vi "datatakersync.vi"() -> ()   [LabVIEW 2013]
doc: "This example demonstrates how to acquire a single buffer of voltage measurements using a DAQmx device.\n\nFor instructions on how to connect your signals to the DAQ device, refer to your device documentation."
uses:
  <vilib>/userdefined/High Color/nirio_resource_hc.ctl
  <vilib>/Utility/error.llb/DialogType.ctl
  <vilib>/FPGAPlugInAG/PCIe-7841R/niLvFpga_Open_PCIe-7841R.vi
  <vilib>/DAQmx/create/channels.llb/DAQmx Create Channel (AI-Voltage-Basic).vi
  <vilib>/DAQmx/configure/timing.llb/DAQmx Timing (Sample Clock).vi
  <vilib>/DAQmx/configure/trigger.llb/DAQmx Start Trigger (Digital Edge).vi
  <vilib>/rvi/interface/nirviOpenFPGA/nirviOpenFPGA.xnode
  fpga/MultiChannelFeed_FPGATarget2_feedbackcooling(_T5hmXv3JUos.lvbitx
  <resource>/objmgr/daqmx.rc
panel:
  in  "sweep time (S)":ext=10.0 format="%.2f"
  in  "sweep stop (Hz)":ext=200.0
  in  "sweep start (Hz)":ext=1.0
  in  "chirp?":bool
  in  "stop (F)":ext=200.0
  in  "start (F)":ext=10.0
  in  "Number of F Steps":i32=20
  in  "dc offset?":bool=TRUE
  in  "volt_div":dbl=200.0
  in  "Set synth?":bool=TRUE
  in  "stop (V)":ext=2.5
  in  "start (V)":ext=2.5
  in  "Number of V Steps":i32=1
  out "error out":errorcluster
  in  "Physical Channel (drive signals)":tag="Dev5/ai0"
  out "Curr threshold":dbl
  in  "Stop threshold":dbl=0.05
  in  "Stop flashing below thresh":bool
  out "Pirani pressure (mbar)":string="0000\r\n"
  out "CC read error":errorcluster={"status"=FALSE, "code"=1073676294, "source"="VISA Read in read_pressure(SubVI).vi->hdf5(SubVI).vi->datataker.vi"}
  out "CC pressure (mbar)":string="4."
  out "Pirani read error":errorcluster={"status"=FALSE, "code"=1073676294, "source"="VISA Read in read_pressure(SubVI).vi->hdf5(SubVI).vi->datataker.vi"}
  in  "# Pulses":i32=3
  in  "Output channel (for flashing)":tag="Dev4/ao0"
  in  "Number of cyles\nbetween flashes":i32=3
  in  "Flash lamp?":bool
  in  "File base name":string="5e-7mbar_xyzcool"
  in  "Delay time between files(s)":dbl caption="Delay Time (s)"
  in  "Num files":i32=100000
  out "Temps (C):":dbl[](array[numeric])=[24.1, 24.6]
  in  "VISA Refnum in":refnum<visa-resource-name>="GPIB0::19::INSTR"
  in  "RIO Device":T1="RIO0::INSTR"
  in  "Directory path":path=path "D:/Data/20140623/Bead1/freq_sweep_finer"
  out "Waveform Graph":dbl[][](graph)
  in  "Number of Samples":i32=500000
  in  "Sample Rate":dbl=5000.0
  in  "Sample Clock Source":tag="/Dev2/PXI_Clk10"
  in  "Terminal Configuration":i32(ring)=-1 items=["default"=-1, "RSE"=10083, "NRSE"=10078, "Differential"=10106, "Pseudodifferential"=12529]
  in  "Max Voltage":dbl=10.0
  in  "Physical Channels (Position signals)":tag="Dev2/ai0:7"
  out "Actual Sample Rate":dbl=5000.0 format="%0.2f"
  # "Channel Settings"
  # "Acquired Data"
  # "Timing Settings"
  # "Flash Lamp Settings"
  # "Pressures and Temperatures"
  # "Logging Settings"
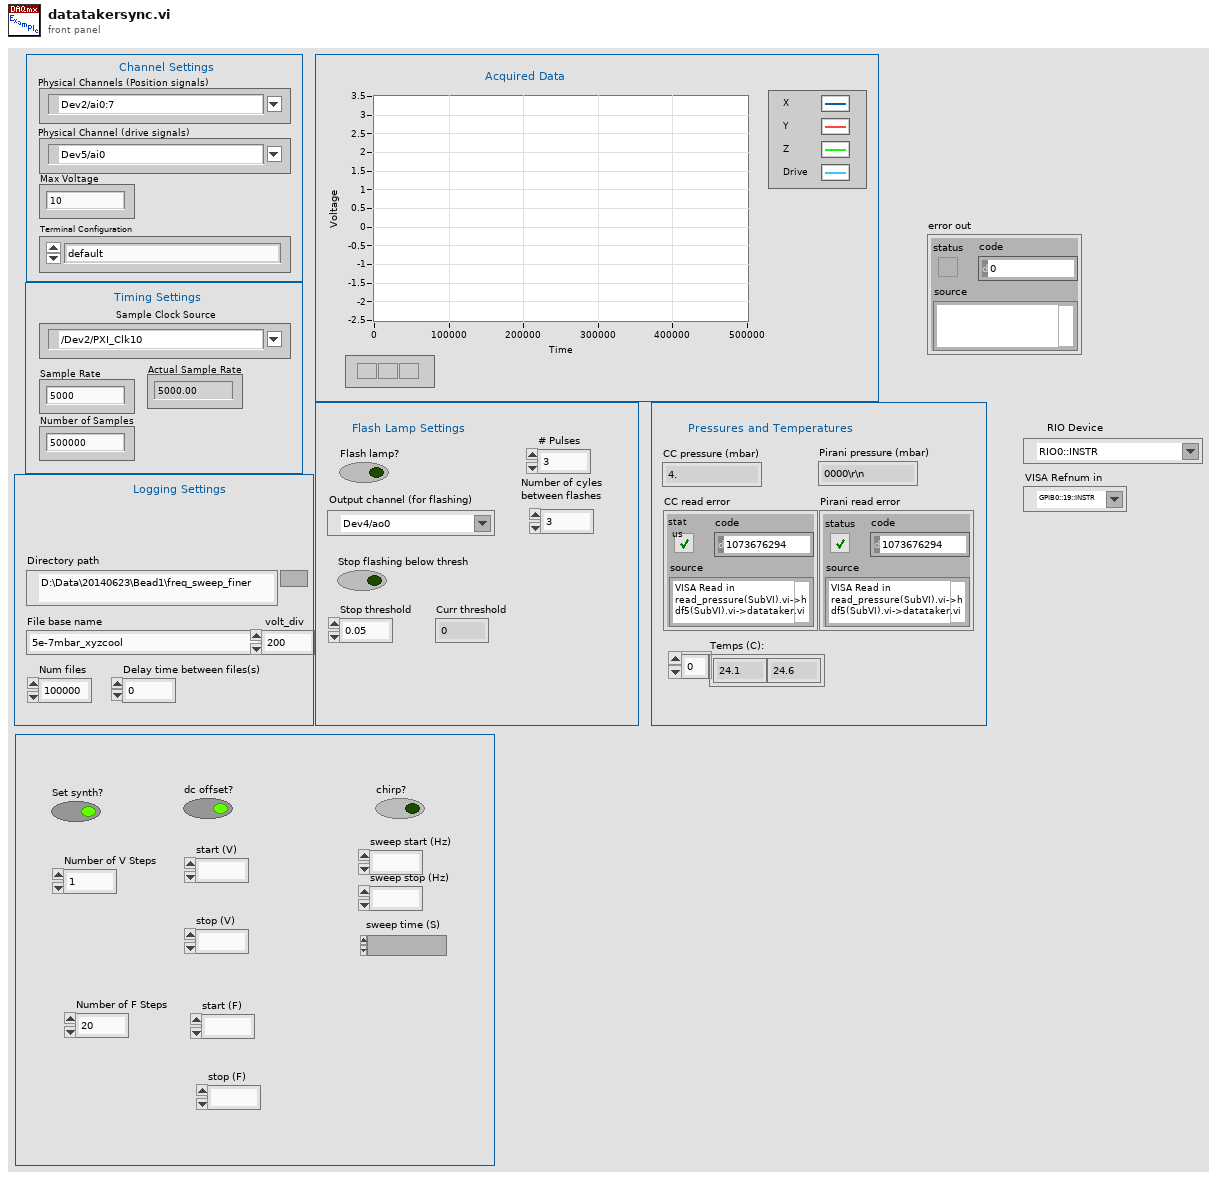
[diagram p1: front panel]
types:
  T1 = typedef "nirio_resource_hc.ctl" = tag
  T2 = typedef "DialogType.ctl" = u16
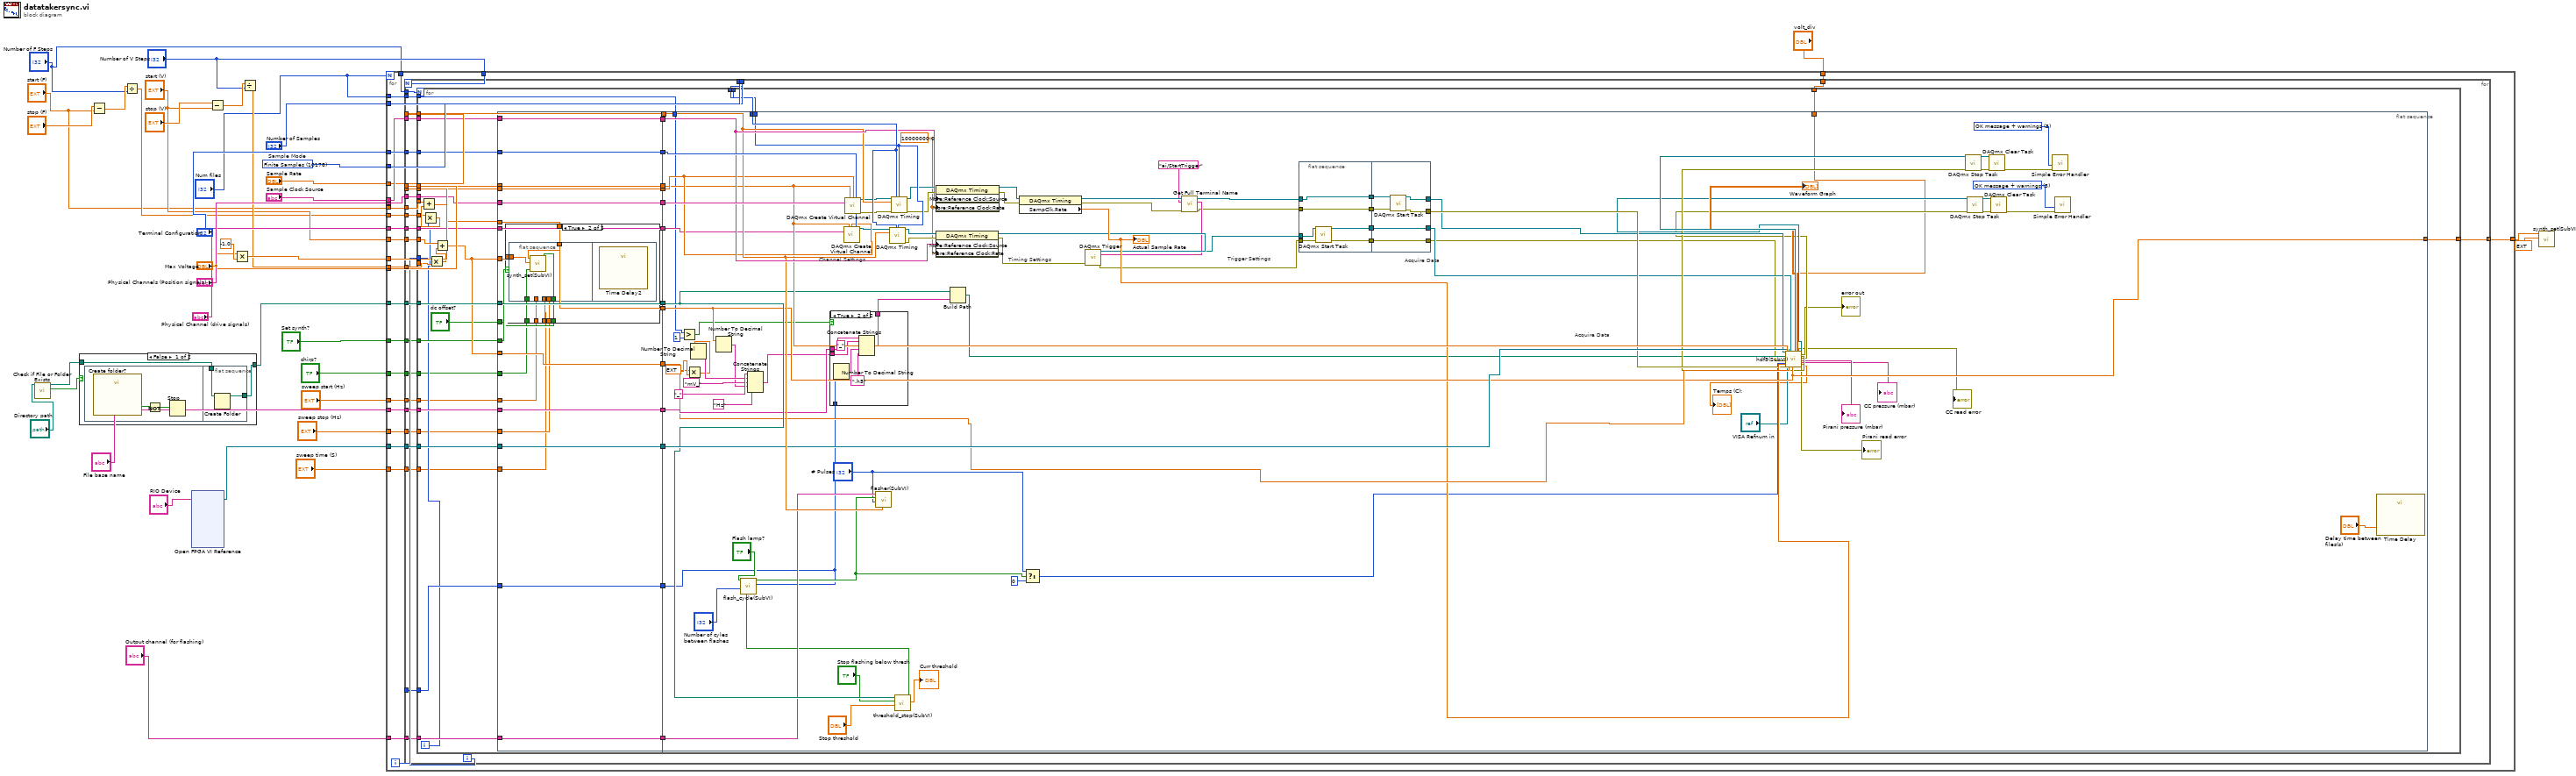
[diagram p0: block diagram]
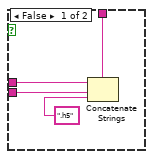
[diagram p3: hidden frame]
diagram:
  w37 = 10178 items=["Finite Samples"=10178, "Continuous Samples"=10123, "Hardware Timed Single Point"=12522]  # Sample Mode
  n1 = call <vilib>:"Check if File or Folder Exists.vi"("path"="Directory path") -> ("file or folder exists?"=w25:bool, "dup path"=w24:path)  [unwired: 8 in, 1 out]
  n2 = case shown="False" w25 {
    tunnel: w24 -> [w39 w44]
    tunnel: [w38 w44] -> w23
    frame False {
      n3 = flat-sequence {
        tunnel: w39 -> [w43]
        tunnel: [w42] -> w38
        frame #0 {
          n4 = call "Create folder?"() -> ("OK"=w41:bool)  [unwired: 18 in, 1 out]
          n5 = Not(x=w41) -> (.not. x?=w40:bool)
          n6 = Stop(stop? (T)=w40) -> ()
        }
        frame #1 {
          n7 = Create Folder(path (use dialog)=w43) -> (created path=w42:path)  [unwired: 2 in, 2 out]
        }
      }
    }
    frame True {
    }
  }
  n8 = Subtract(x="stop (F)", y="start (F)") -> (x-y=w9:ext)
  n9 = Divide(x=w9, y="Number of F Steps") -> (x/y=w8:ext)
  n10 = xnode "Open FPGA VI Reference"("resource name"="RIO Device") -> ("FPGA VI Reference Out"=w27:refnum<k20>)  [unwired: 1 in, 1 out]
  n11 = Subtract(x="stop (V)", y="start (V)") -> (x-y=w18:ext)
  n12 = Multiply(x="Max Voltage", y=-1.0) -> (x*y=w30:dbl)
  n13 = Divide(x=w18, y="Number of V Steps") -> (x/y=w16:ext)
  n14 = for {
    N: "Num files" -> [_]
    tunnel: w37 -> [w72]
    tunnel: "Physical Channels (Position signals)" -> [w71]
    tunnel: "Terminal Configuration" -> [w70]
    tunnel: "Sample Clock Source" -> [w69]
    tunnel: "Sample Rate" -> [w68]
    tunnel: "Number of Samples" -> [w67]
    tunnel: w30 -> [w66]
    tunnel: "Max Voltage" -> [w65]
    tunnel: w27 -> [w64]
    tunnel: w23 -> [w63]
    tunnel: "File base name" -> [w62]
    tunnel: "Output channel (for flashing)" -> [w61]
    tunnel: "Physical Channel (drive signals)" -> [w60]
    tunnel: "Number of V Steps" -> [w59]
    tunnel: w16 -> [w58]
    tunnel: "start (V)" -> [w57]
    tunnel: [w56] -> w6
    tunnel: "Num files" -> [w54]
    tunnel: "Set synth?" -> [w53]
    tunnel: "volt_div" -> [w52]
    tunnel: w8 -> [w51]
    tunnel: "start (F)" -> [w50]
    tunnel: "Number of F Steps" -> [w49]
    tunnel: "chirp?" -> [w48]
    tunnel: "sweep start (Hz)" -> [w47]
    tunnel: "sweep stop (Hz)" -> [w46]
    tunnel: "sweep time (S)" -> [w45]
    i -> [w55]
    n15 = for {
      N: w59 -> [_]
      tunnel: w72 -> [w100]
      tunnel: w71 -> [w99]
      tunnel: w70 -> [w98]
      tunnel: w69 -> [w97]
      tunnel: w68 -> [w96]
      tunnel: w67 -> [w95]
      tunnel: w66 -> [w94]
      tunnel: w65 -> [w93]
      tunnel: w64 -> [w92]
      tunnel: w63 -> [w91]
      tunnel: w62 -> [w90]
      tunnel: w61 -> [w89]
      tunnel: w60 -> [w88]
      tunnel: w58 -> [w87]
      tunnel: w57 -> [w86]
      tunnel: [w85] -> w56
      tunnel: w55 -> [w83]
      tunnel: w54 -> [w82]
      tunnel: w53 -> [w81]
      tunnel: w52 -> [w80]
      tunnel: w51 -> [w79]
      tunnel: w50 -> [w78]
      tunnel: w49 -> [w77]
      tunnel: w48 -> [w76]
      tunnel: w47 -> [w75]
      tunnel: w46 -> [w74]
      tunnel: w45 -> [w73]
      i -> [w84]
      n16 = for {
        N: w77 -> [_]
        tunnel: w100 -> [w133]
        tunnel: w99 -> [w132]
        tunnel: w98 -> [w131]
        tunnel: w97 -> [w130]
        tunnel: w96 -> [w129]
        tunnel: w95 -> [w128]
        tunnel: w94 -> [w127]
        tunnel: w93 -> [w126]
        tunnel: w92 -> [w125]
        tunnel: w91 -> [w124]
        tunnel: w90 -> [w123]
        tunnel: w89 -> [w122]
        tunnel: w88 -> [w121]
        tunnel: w87 -> [w120]
        tunnel: w86 -> [w118]
        tunnel: [w116] -> w85
        tunnel: w84 -> [w115]
        tunnel: w83 -> [w114]
        tunnel: w82 -> [w113]
        tunnel: w81 -> [w112]
        tunnel: w80 -> [w111]
        tunnel: w79 -> [w107]
        tunnel: w78 -> [w106]
        tunnel: w76 -> [w104]
        tunnel: w75 -> [w103]
        tunnel: w74 -> [w102]
        tunnel: w73 -> [w101]
        i -> [w105]
        n17 = Multiply(x=w107, y=w105) -> (x*y=w108:ext)
        n18 = Add(x=w106, y=w108) -> (x+y=w109:ext)
        n19 = Multiply(x=w115, y=w120) -> (x*y=w119:ext)
        n20 = Add(x=w118, y=w119) -> (x+y=w117:ext)
        n21 = flat-sequence {
          tunnel: w121 -> [w157]
          tunnel: w122 -> [w158]
          tunnel: w123 -> [w159]
          tunnel: w124 -> [w160]
          tunnel: w125 -> [w161]
          tunnel: w126 -> [w162]
          tunnel: w127 -> [w163]
          tunnel: w130 -> [w164]
          tunnel: w131 -> [w165]
          tunnel: w132 -> [w166]
          tunnel: [w166] -> w146
          tunnel: [w165] -> w145
          tunnel: [w164] -> w144
          tunnel: [w163] -> w143
          tunnel: [w162] -> w142
          tunnel: [w161] -> w141
          tunnel: [w160] -> w140
          tunnel: [w159] -> w139
          tunnel: [w158] -> w138
          tunnel: [w157] -> w137
          tunnel: w109 -> [w155]
          tunnel: w117 -> [w156]
          tunnel: [w155] -> w136
          tunnel: w117 -> [w154]
          tunnel: [w154] -> w135
          tunnel: w114 -> [w153]
          tunnel: [w153] -> w134
          tunnel: w112 -> [w152]
          tunnel: "dc offset?" -> [w151]
          tunnel: w104 -> [w150]
          tunnel: w103 -> [w149]
          tunnel: w102 -> [w148]
          tunnel: w101 -> [w147]
          tunnel: w133 -> [w267]
          tunnel: w129 -> [w263]
          tunnel: w128 -> [w262]
          tunnel: w146 -> [w266]
          tunnel: w145 -> [w265]
          tunnel: w144 -> [w264]
          tunnel: w143 -> [w261]
          tunnel: w142 -> [w260]
          tunnel: w141 -> [w259]
          tunnel: w140 -> [w258]
          tunnel: w139 -> [w257]
          tunnel: w138 -> [w256]
          tunnel: w137 -> [w255]
          tunnel: w136 -> [w253]
          tunnel: w135 -> [w254]
          tunnel: [w253] -> w116
          tunnel: w134 -> [w180]
          tunnel: w113 -> [w179]
          tunnel: w111 -> [w178]
          frame #0 {
            n22 = case shown="True" w152 {
              tunnel: w156 -> [_ w173]
              tunnel: w155 -> [_ w172]
              tunnel: w151 -> [_ w171]
              tunnel: w150 -> [_ w170]
              tunnel: w149 -> [_ w169]
              tunnel: w148 -> [_ w168]
              tunnel: w147 -> [_ w167]
              frame False {
              }
              frame True {
                n23 = flat-sequence {
                  tunnel: w173 -> [w177]
                  tunnel: w172 -> [w176]
                  tunnel: w171 -> [w175]
                  tunnel: w170 -> [w174]
                  tunnel: w169 -> [_]
                  tunnel: w168 -> [_]
                  tunnel: w167 -> [_]
                  frame #0 {
                    n24 = call "synth_set(SubVI).vi"("dc offset?"=w175, "chirp?"=w174, "amplitude (V)"=w177, "frequency (Hz)"=w176) -> ()  [unwired: 6 in, 2 out]
                  }
                  frame #1 {
                    n25 = call "Time Delay2"() -> ()  [unwired: 11 in, 1 out]
                  }
                }
              }
            }
          }
          frame #1 {
            w198 = 10000000.0 ("RefClk.Rate")
            w201 = T2 3 items=["no dialog", "OK message", "continue or stop message", "OK message + warnings", "continue/stop + warnings"] ("type of dialog (OK msg:1)")
            w245 = T2 3 items=["no dialog", "OK message", "continue or stop message", "OK message + warnings", "continue/stop + warnings"] ("type of dialog (OK msg:1)")
            # "Acquire Data"
            # "Acquire Data"
            # "Trigger Settings"
            # "Timing Settings"
            # "Channel Settings"
            n26 = Greater?(x=w179, y=1) -> (0:w237:bool)
            n27 = Multiply(x=ext 1000.0, y=w254) -> (x*y=w181:ext)
            n28 = Number To Decimal String(number=w181) -> (decimal integer string=w187:string)  [unwired: 1 in]
            n29 = Number To Decimal String(number=w253) -> (decimal integer string=w185:string)  [unwired: 1 in]
            n30 = Concatenate Strings("_" ("string"), w187, "mV_" ("string"), w185, "Hz" ("string")) -> (w183:string)
            n31 = case shown="True" w237 {
              tunnel: w180 -> [_ w288]
              tunnel: [w282 w286] -> w235
              tunnel: w183 -> [w281 w284]
              tunnel: w257 -> [w280 w285]
              frame False {
                n32 = Concatenate Strings(w280, w281, ".h5" ("string")) -> (w282:string)
              }
              frame True {
                n33 = Number To Decimal String(number=w288) -> (decimal integer string=w289:string)  [unwired: 1 in]
                n34 = Concatenate Strings(w285, w284, "_" ("string"), w289, ".h5" ("string")) -> (w286:string)
              }
            }
            n35 = call-poly <vilib>:"DAQmx Create Virtual Channel.vi"("maximum value"=w260, "minimum value"=w261, "input terminal configuration"=w265, "physical channels"=w255) -> ("task out"=w224:refnum<k21>)  [unwired: 10 in, 1 out]
            n36 = call-poly <vilib>:"DAQmx Create Virtual Channel.vi"("maximum value"=w260, "minimum value"=w261, "input terminal configuration"=w265, "physical channels"=w266) -> ("task out"=w226:refnum<k21>, "error out"=w225:errorcluster)  [unwired: 10 in]
            n37 = call-poly <vilib>:"DAQmx Timing.vi"("task/channels in"=w224, "sample mode"=w267, "samples per channel"=w262, "rate"=w263) -> ("task out"=w221:refnum<k21>, "error out"=w220:errorcluster)  [unwired: 10 in]
            n38 = call-poly <vilib>:"DAQmx Timing.vi"("task/channels in"=w226, "sample mode"=w267, "samples per channel"=w262, "rate"=w263, "error in"=w225) -> ("task out"=w223:refnum<k21>, "error out"=w222:errorcluster)  [unwired: 9 in]
            n39 = call "threshold_stop(SubVI).vi"("Stop threshold"="Stop threshold", "Stop flashing below thresh"="Stop flashing below thresh", "dup path"=w258) -> ("Curr threshold"=→"Curr threshold":dbl, "Boolean"=w231:bool)  [unwired: 7 in]
            n40 = call "flash_cycle(SubVI).vi"("Boolean in"=w231, "Number of cyles\nbetween flashes"="Number of cyles\nbetween flashes", "Numeric"=w180, "Flash lamp?"="Flash lamp?") -> ("Boolean out"=w230:bool)  [unwired: 7 in]
            n41 = call "flasher(SubVI).vi"("Sample Rate"=w263, "# Pulses"="# Pulses", "Boolean"=w230, "Output channel (for flashing)"=w256) -> ()  [unwired: 8 in]
            n42 = property class="DAQmx Timing"(reference=w221, error in=w220, "More:Reference Clock:Source"=w264, "More:Reference Clock:Rate"=w198) -> (reference out=w214:refnum<k21>, error out=w213:errorcluster)
            n43 = property class="DAQmx Timing"(reference=w223, error in=w222, "More:Reference Clock:Source"=w264, "More:Reference Clock:Rate"=w198) -> (reference out=w219:refnum<k21>, error out=w218:errorcluster)
            n44 = Build Path(base path=w258, name or relative path=w235) -> (appended path=w236:path)
            n45 = property class="DAQmx Timing"(reference=w219, error in=w218) -> (reference out=w217:refnum<k21>, error out=w215:errorcluster, "SampClk.Rate"=w244:dbl)
            "Actual Sample Rate" <- w244
            n46 = Select(t="# Pulses", s=w230, f=0) -> (s? t:f=w227:i32)
            n47 = call "Get Full Terminal Name.vi"("error in (no error)"=w215, "Local Terminal Name"="ai/StartTrigger", "task/channels in"=w217) -> ("error out"=w210:errorcluster, "Terminal Name with Device Prefix"=w212:tag, "task out"=w211:refnum<k21>)  [unwired: 6 in]
            n48 = call-poly <vilib>:"DAQmx Trigger.vi"("task/channels in"=w214, "source"=w212, "error in"=w213) -> ("task out"=w209:refnum<k21>, "error out"=w208:errorcluster)  [unwired: 11 in]
            n49 = flat-sequence {
              tunnel: w211 -> [w271]
              tunnel: w210 -> [w270]
              tunnel: w209 -> [w273]
              tunnel: w208 -> [w272]
              tunnel: [w271] -> w252
              tunnel: [w270] -> w251
              tunnel: [w269] -> w250
              tunnel: [w268] -> w249
              tunnel: [w278] -> w242
              tunnel: [w276] -> w243
              tunnel: w252 -> [w279]
              tunnel: w251 -> [w277]
              tunnel: [w275] -> w207
              tunnel: w250 -> [w275]
              tunnel: [w274] -> w206
              tunnel: w249 -> [w274]
              frame #0 {
                n50 = call <vilib>:"DAQmx Start Task.vi"("task/channels in"=w273, "error in"=w272) -> ("task out"=w269:refnum<k21>, "error out"=w268:errorcluster)  [unwired: 12 in]
              }
              frame #1 {
                n51 = call <vilib>:"DAQmx Start Task.vi"("task/channels in"=w279, "error in"=w277) -> ("task out"=w278:refnum<k21>, "error out"=w276:errorcluster)  [unwired: 12 in]
              }
            }
            n52 = call "hdf5(SubVI).vi"("Refnum in"=w242, "VISA Refnum in"="VISA Refnum in", "appended path"=w236, "Max Voltage"=w260, "error out 3"=w206, "f"=w227, "SampClk.Rate"=w244, "error in (no error)"=w243, "FPGA VI Reference Out"=w259, "drive_amplitude"=w254, "task in"=w207, "drive_freq"=w253, "volt_div"=w178) -> ("task out 4"=w241:refnum<k21>, "Array"=→"Waveform Graph":dbl[][], "CC read error"=→"CC read error":errorcluster, "Refnum out"=w200:refnum<k21>, 21:"error out"=→"error out":errorcluster, "error out 4"=w240:errorcluster, "error out 2"=w199:errorcluster, "Pirani pressure (mbar)"=→"Pirani pressure (mbar)":string, "CC pressure (mbar)"=→"CC pressure (mbar)":string, "Temps (C):"=→"Temps (C):":dbl[], 27:"error out"=→"Pirani read error":errorcluster)  [unwired: 4 in]
            n53 = call <vilib>:"DAQmx Stop Task.vi"("task/channels in"=w241, "error in"=w240) -> ("task out"=w247:refnum<k21>, "error out"=w246:errorcluster)  [unwired: 12 in]
            n54 = call <vilib>:"DAQmx Stop Task.vi"("task/channels in"=w200, "error in"=w199) -> ("task out"=w203:refnum<k21>, "error out"=w202:errorcluster)  [unwired: 12 in]
            n55 = call <vilib>:"DAQmx Clear Task.vi"("task in"=w247, "error in"=w246) -> ("error out"=w248:errorcluster)  [unwired: 13 in]
            n56 = call <vilib>:"DAQmx Clear Task.vi"("task in"=w203, "error in"=w202) -> ("error out"=w204:errorcluster)  [unwired: 13 in]
            n57 = call <vilib>:"Simple Error Handler.vi"("type of dialog (OK msg:1)"=w245, "error in (no error)"=w248) -> ()  [unwired: 3 in, 5 out]
            n58 = call <vilib>:"Simple Error Handler.vi"("type of dialog (OK msg:1)"=w201, "error in (no error)"=w204) -> ()  [unwired: 3 in, 5 out]
            n59 = call "Time Delay"("Delay Time (s)"="Delay time between files(s)") -> ()  [unwired: 10 in, 1 out]
          }
        }
      }
    }
  }
  n60 = call "synth_set(SubVI).vi"("amplitude (V)"=ext 0.00099999999999999999996, "frequency (Hz)"=w6) -> ()  [unwired: 8 in, 2 out]
